vi "UHR-Fleezers Control (host) - 12.6.1.vi"() -> ()   [LabVIEW 2012] (continued)
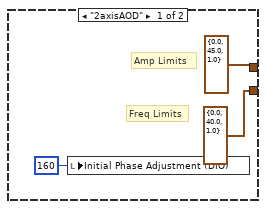
[diagram p2: hidden frame]
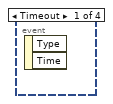
[diagram p3: hidden frame]
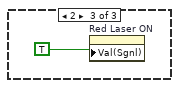
[diagram p6: hidden frame]
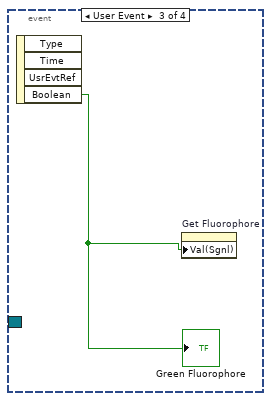
[diagram p7: hidden frame]
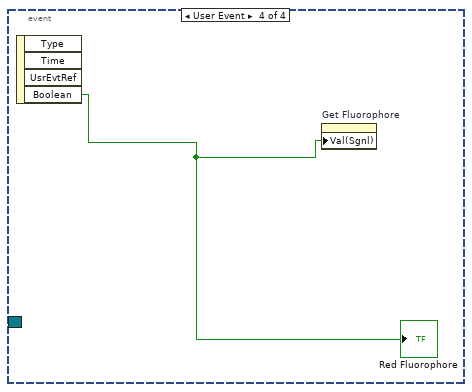
[diagram p8: hidden frame]
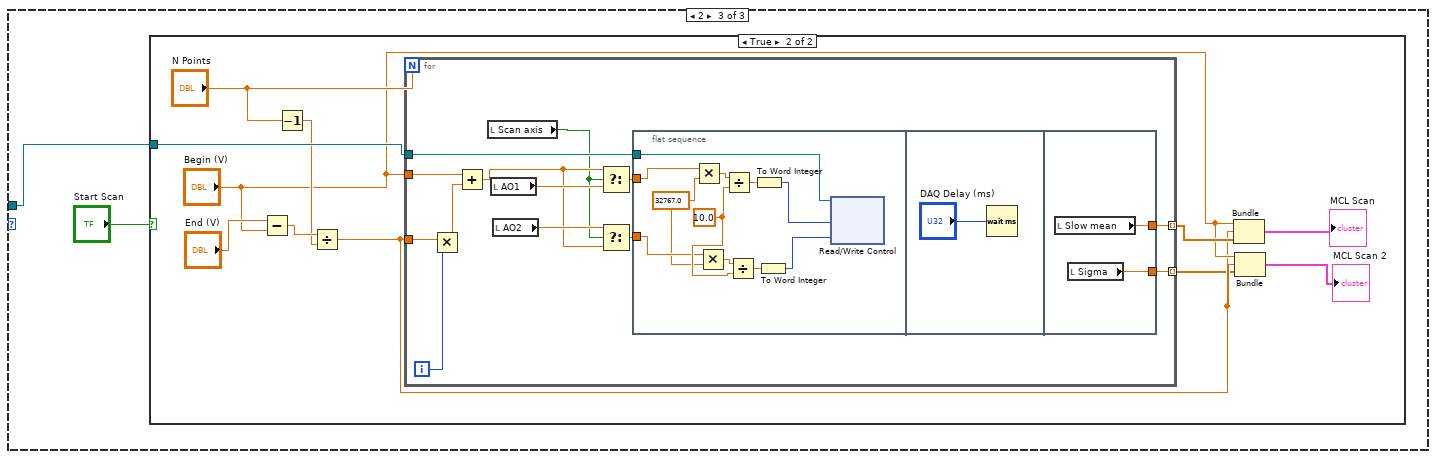
[diagram p10: hidden frame]
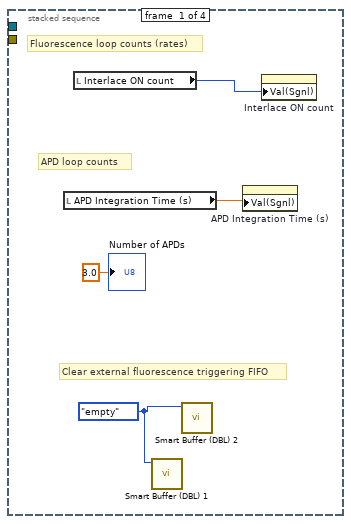
[diagram p12: hidden frame]
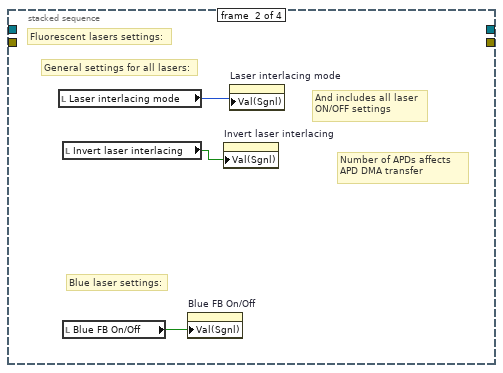
[diagram p13: hidden frame]
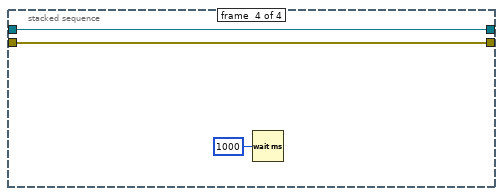
[diagram p14: hidden frame]
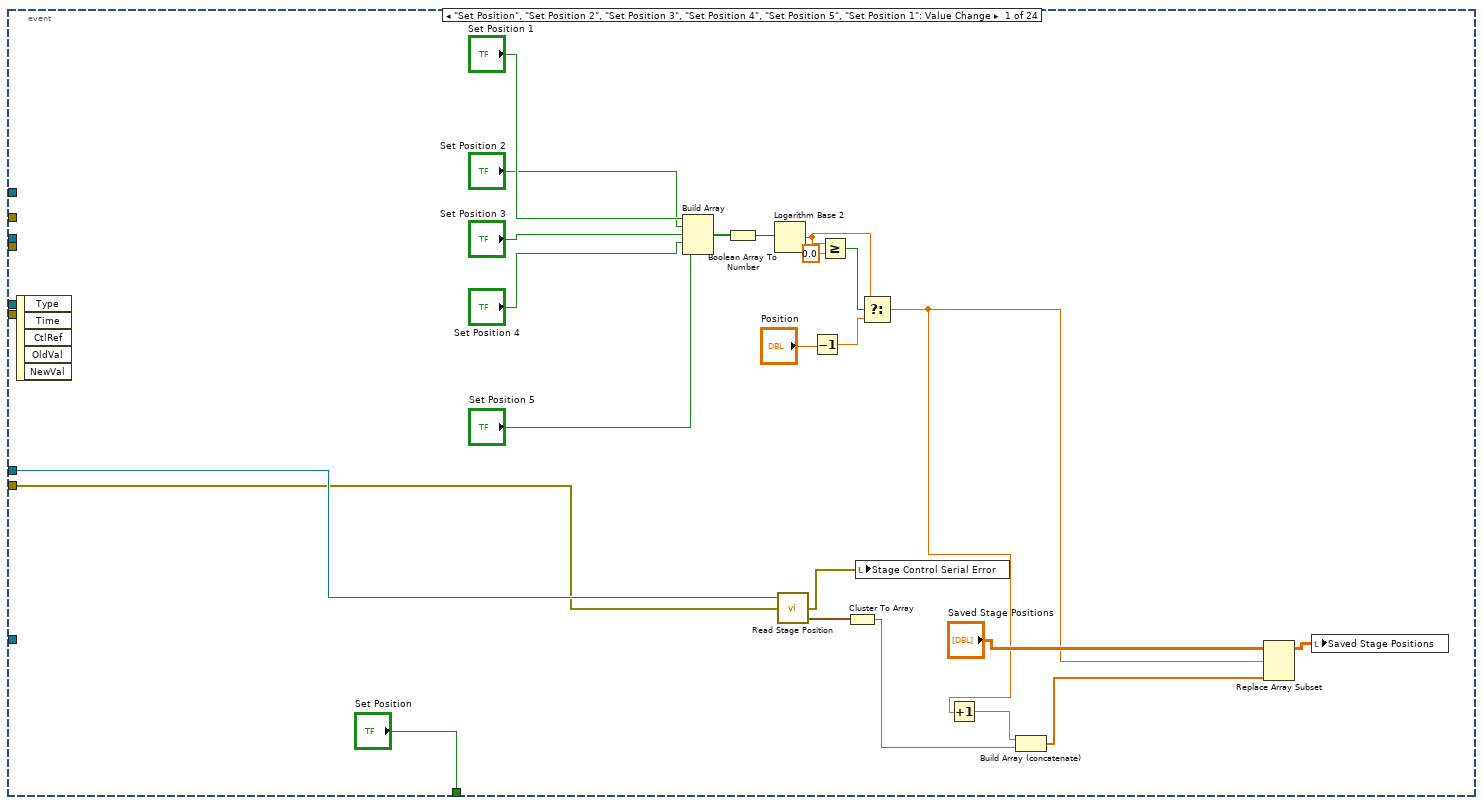
[diagram p16: hidden frame]
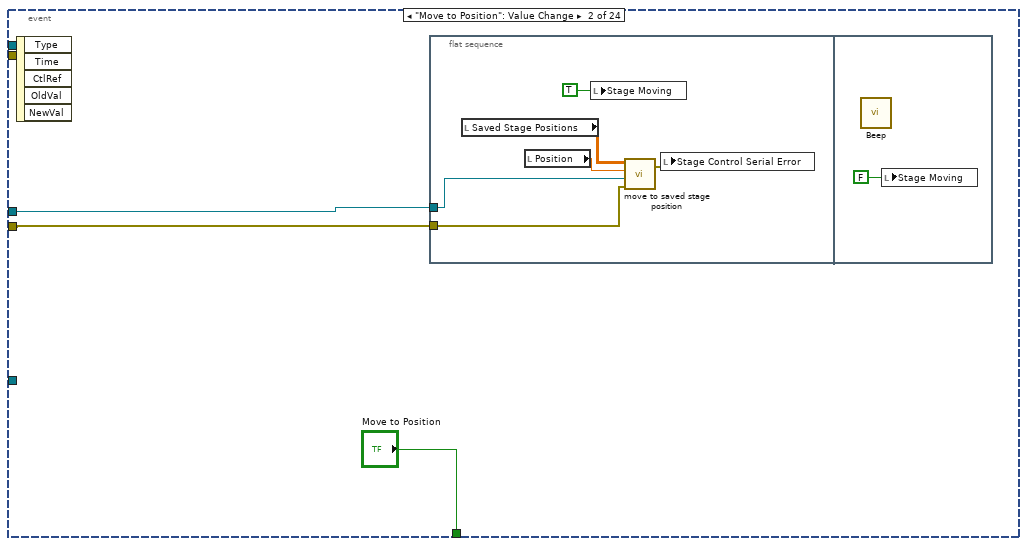
[diagram p17: hidden frame]
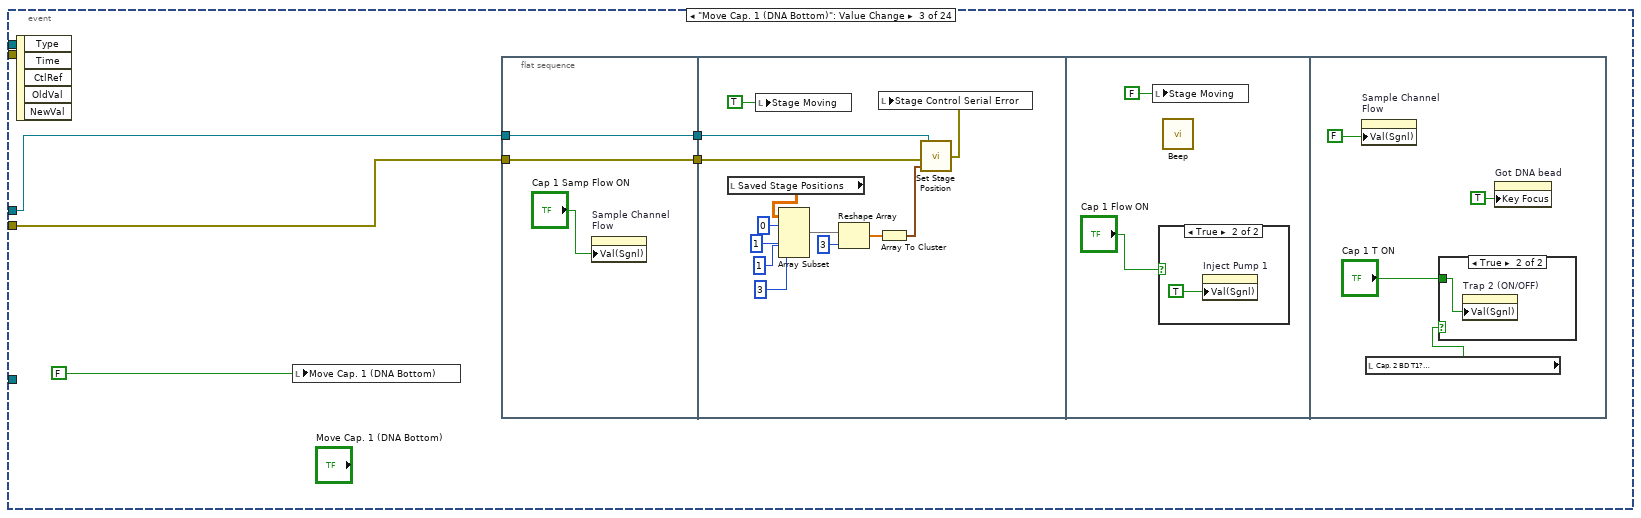
[diagram p18: hidden frame]
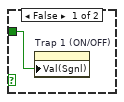
[diagram p20: hidden frame]
            n2987 = Build Array (concatenate)(w4589, w4590, w4587) -> (w4562:dbl[])
            n2988 = case "If fluorescence data to be saved" shown="True" w4579 {
              tunnel: w4563 -> [_ w4657]
              tunnel: [refnum<k0> refnum w4637] -> w4580
              frame False {
              }
              frame True {
                w4636 = 0.0
                n2989 = local read "APD Integration Time (s)"() -> (w4642:dbl)
                n2990 = local read "N APD Samp/step"() -> (w4635:dbl)
                n2991 = local read "Number of APDs"() -> (w4634:u8)
                n2992 = Path To String(path=w4657) -> (string=w4656:string)
                n2993 = String Length(string=w4656) -> (length=w4655:i32)
                n2994 = Subtract(x=w4655, y=4) -> (x-y=w4653:i32)
                n2995 = String Subset(string=w4656, length (rest)=w4653) -> (substring=w4652:string)  [unwired: 1 out]
                n2996 = Build Array(w4642, w4635, w4634, w4636, w4636, w4636, w4636, w4636) -> (w4639:dbl[])
                n2997 = Concatenate Strings(w4652, "_fl.dat" ("string")) -> (w4650:string)
                n2998 = Array Size(array=w4639) -> (size(s)=w4641:i32)
                n2999 = String To Path(string=w4650) -> (path=w4646:path)
                n3000 = Open/Create/Replace File(file path (use dialog)=w4646, operation (0:open)=T29."create", access (0:read/write)=enum16{"read/write", "read-only", "write-only"}."write-only") -> (refnum out=w4647:refnum<file>)  [unwired: 1 in, 4 out]
                n3001 = Deny Access(7:w4647) -> (3:w4643:refnum<file>)  [unwired: 1 in, 2 out]
                n3002 = To Double Precision Float(number=w4641) -> (double precision float=w4640:dbl)
                n3003 = Build Array (concatenate)(w4640, w4639) -> (w4638:dbl[])
                n3004 = Write to Binary File(file (use dialog)=w4643, data=w4638, 5:FALSE ("prepend array or string size? (T)"), 9:T28."big-endian, network order" ("byte order (0:big-endian, network order)")) -> (refnum out=w4637:refnum<file>)  [unwired: 1 in, 3 out]
              }
            }
            n3005 = case shown="True" w4567 {
              tunnel: w4563 -> [_ w4618]
              tunnel: [refnum<k0> refnum w4617] -> w4568
              frame False {
              }
              frame True {
                w4613 = 0.0 ("element")
                n3006 = Path To String(path=w4618) -> (string=w4632:string)
                n3007 = Build Array(w4613, w4613, w4613, w4613, w4613, w4613, w4613, w4613) -> (w4614:dbl[])
                n3008 = String Length(string=w4632) -> (length=w4631:i32)
                n3009 = Subtract(x=w4631, y=4) -> (x-y=w4629:i32)
                n3010 = Array Size(array=w4614) -> (size(s)=w4616:i32)
                n3011 = String Subset(string=w4632, length (rest)=w4629) -> (substring=w4628:string)  [unwired: 1 out]
                n3012 = To Double Precision Float(number=w4616) -> (double precision float=w4615:dbl)
                n3013 = Concatenate Strings(w4628, "_pos.dat" ("string")) -> (w4626:string)
                n3014 = Build Array (concatenate)(w4615, w4614) -> (w4612:dbl[])
                n3015 = String To Path(string=w4626) -> (path=w4622:path)
                n3016 = Open/Create/Replace File(file path (use dialog)=w4622, operation (0:open)=T29."create", access (0:read/write)=enum16{"read/write", "read-only", "write-only"}."write-only") -> (refnum out=w4623:refnum<file>)  [unwired: 1 in, 4 out]
                n3017 = Deny Access(7:w4623) -> (3:w4619:refnum<file>)  [unwired: 1 in, 2 out]
                n3018 = Write to Binary File(file (use dialog)=w4619, data=w4612, 5:FALSE ("prepend array or string size? (T)"), 9:T28."big-endian, network order" ("byte order (0:big-endian, network order)")) -> (refnum out=w4617:refnum<file>)  [unwired: 1 in, 3 out]
              }
            }
            n3019 = Write to Binary File(file (use dialog)=w4603, data=w4562, 5:w4585, 9:w4584) -> (refnum out=w4586:refnum<file>)  [unwired: 1 in, 3 out]
            n3020 = Write to Binary File(file (use dialog)=w4586, data="Comment (data description)", 5:w4585, 9:w4584) -> (refnum out=w4583:refnum<file>)  [unwired: 1 in, 3 out]
            n3021 = local read "connection reference"() -> (w4565:T17)
            n3022 = Bundle("Comment (data description)"="Comment (data description)", "Channel 1 Buffer"="Channel 1 Buffer", "Channel 2 Buffer"="Channel 2 Buffer", "Channel 3 Buffer"="Channel 3 Buffer", "Title"="Title", "DNA Construct"="DNA Construct", "Bead diameter"="Bead diameter", "Name"="Name") -> (w4553:T47)  [unwired: 1 in]
            n3023 = call "MattFileCreator-v9.vi"("Comments"=w4553, "Input Array"=w4562, "File path"=w4563, "table"="labview", "connection reference"=w4565) -> ("connection reference out"=w4564:T17)  [unwired: 5 in, 1 out]
            n3024 = local write "connection reference"(w4564) -> ()
          }
        }
        n3025 = feedback-in #27(w4513) -> ()
        n3026 = feedback-in #28(w4540) -> ()
        n3027 = feedback-in #29(w4512) -> ()
        n3028 = feedback-in #30(w4523) -> ()
        n3029 = feedback-in #31(w4526) -> ()
        n3030 = feedback-in #32(w4539) -> ()
        n3031 = feedback-in #33(w4529) -> ()
      }
      frame #1 {
        n3032 = local read "Saving..."() -> (w4783:bool)
        n3033 = case shown="True" w4783 {
          tunnel: w4787 -> [_ w4798]
          tunnel: w4786 -> [_ w4812]
          tunnel: w4785 -> [_ w4808]
          tunnel: w4784 -> [_ w4807]
          tunnel: w4782 -> [_ w4806]
          tunnel: w4781 -> [_ w4801]
          tunnel: w4780 -> [_ w4800]
          tunnel: w4779 -> [_ w4799]
          tunnel: w4778 -> [_ w4797]
          tunnel: w4777 -> [_ w4795]
          tunnel: w4776 -> [_ w4794]
          tunnel: w4775 -> [_ w4793]
          tunnel: w4774 -> [_ w4792]
          tunnel: w4773 -> [_ w4791]
          tunnel: w4772 -> [_ w4790]
          tunnel: w4771 -> [_ w4789]
          tunnel: w4770 -> [_ w4788]
          frame False {
          }
          frame True {
            n3034 = Multiply(x=w4798, y=w4797) -> (x*y=→"Time (s)":dbl)
            n3035 = Less Or Equal?(x=w4798, y=w4806) -> (x <= y?=w4810:bool)
            n3036 = Or(x="Stop Saving", y="Abort save 2") -> (x .or. y?=w4802:bool)
            n3037 = Not(x=w4802) -> (.not. x?=w4811:bool)
            n3038 = And(x=w4810, y=w4811) -> (x .and. y?=w4809:bool)
            n3039 = case shown="True" w4809 {
              tunnel: w4812 -> [w4819 w4910]
              tunnel: [0.0 w4913] -> w4805
              tunnel: w4798 -> [_ w4911]
              tunnel: w4806 -> [_ w4912]
              tunnel: w4808 -> [_ w4907]
              tunnel: w4807 -> [_ _]
              tunnel: w4801 -> [w4817 w4900]
              tunnel: w4800 -> [w4816 w4901]
              tunnel: w4799 -> [_ w4899]
              tunnel: w4795 -> [_ w4898]
              tunnel: w4794 -> [_ w4822]
              tunnel: w4793 -> [_ w4891]
              tunnel: w4792 -> [_ w4838]
              tunnel: w4791 -> [w4813 w4855]
              tunnel: w4790 -> [w4814 w4854]
              tunnel: w4789 -> [_ w4851]
              tunnel: w4788 -> [_ w4849]
              frame False {
                w4815 = FALSE
                n3040 = Close File(refnum=w4819) -> ()  [unwired: 1 in, 2 out]
                n3041 = case shown="True" w4816 {
                  tunnel: w4817 -> [_ w4821]
                  frame False {
                  }
                  frame True {
                    n3042 = Close File(refnum=w4821) -> ()  [unwired: 1 in, 2 out]
                  }
                }
                n3043 = case shown="True" w4813 {
                  tunnel: w4814 -> [_ w4820]
                  frame False {
                  }
                  frame True {
                    n3044 = Close File(refnum=w4820) -> ()  [unwired: 1 in, 2 out]
                  }
                }
                n3045 = local write "Raster Scanning..."(w4815) -> ()
                n3046 = local write "Calibrating Trap..."(w4815) -> ()
                n3047 = call <vilib>:"Beep.vi"() -> ()  [unwired: 3 in, 9 out]
                n3048 = local write "Stop Saving"(w4815) -> ()
                "Saving..." <- w4815
              }
              frame True {
                n3049 = local read "Calibrating Trap..."() -> (w4902:bool)
                n3050 = case "Write fl. data" shown="True" w4901 {
                  tunnel: w4900 -> [_ w4936]
                  tunnel: w4899 -> [_ w4935]
                  frame False {
                  }
                  frame True {
                    n3051 = Write to Binary File(file (use dialog)=w4936, data=w4935, 5:FALSE ("prepend array or string size? (T)"), 9:T28."big-endian, network order" ("byte order (0:big-endian, network order)")) -> ()  [unwired: 1 in, 4 out]
                  }
                }
                n3052 = Greater?(x="Save ave N", y=1.0) -> (0:w4905:bool)
                n3053 = Not(x=w4902) -> (.not. x?=w4904:bool)
                n3054 = And(x=w4904, y=w4905) -> (x .and. y?=w4852:bool)
                n3055 = case shown="True" w4852 {
                  tunnel: w4851 -> [w4916 w4927]
                  tunnel: [w4916 w4919] -> w4850
                  tunnel: "Save ave N" -> [_ w4920]
                  frame False {
                  }
                  frame True {
                    w4917 = 2 ("dimension size")
                    n3056 = Array Size(array=w4927) -> (size(s)=w4921:i32)
                    n3057 = Divide(x=w4921, y=w4917) -> (x/y=w4925:dbl)
                    n3058 = Reshape Array(w4927, w4925, w4917) -> (w4926:u64[][])
                    n3059 = Transpose 2D Array(2D array=w4926) -> (transposed array=w4924:u64[][])
                    n3060 = for {
                      tunnel: w4924 -> [w4929] mode=indexing
                      tunnel: [w4928] -> w4918 mode=indexing
                      tunnel: w4920 -> [w4930]
                      workers-P: _ -> [_]
                      n3061 = call "downsample 1D array - U64.vi"("Ave N"=w4930, "Array In"=w4929) -> ("Array Out"=w4928:u64[])  [unwired: 1 in]
                    }
                    n3062 = Transpose 2D Array(2D array=w4918) -> (transposed array=w4923:u64[][])
                    n3063 = Divide(x=w4921, y=w4920) -> (x/y=w4922:dbl)
                    n3064 = Reshape Array(w4923, w4922) -> (w4919:u64[])
                  }
                }
                n3065 = case shown="True" w4852 {
                  tunnel: w4907 -> [w4939 w4951]
                  tunnel: [w4939 w4943] -> w4903
                  tunnel: "Save ave N" -> [_ w4944]
                  tunnel: w4898 -> [_ w4942]
                  frame False {
                  }
                  frame True {
                    n3066 = Array Size(array=w4951) -> (size(s)=w4945:i32)
                    n3067 = Array Size(array=w4942) -> (size(s)=w4941:i32)
                    n3068 = Divide(x=w4945, y=w4941) -> (x/y=w4949:dbl)
                    n3069 = Reshape Array(w4951, w4949, w4941) -> (w4950:i16[][])
                    n3070 = Transpose 2D Array(2D array=w4950) -> (transposed array=w4948:i16[][])
                    n3071 = for {
                      tunnel: w4948 -> [w4954] mode=indexing
                      tunnel: [w4953] -> w4940 mode=indexing
                      tunnel: w4944 -> [w4952]
                      workers-P: _ -> [_]
                      n3072 = call "downsample 1D array - I16.vi"("Ave N"=w4952, "Array In"=w4954) -> ("Array Out"=w4953:i16[])  [unwired: 1 out]
                    }
                    n3073 = Transpose 2D Array(2D array=w4940) -> (transposed array=w4947:i16[][])
                    n3074 = Divide(x=w4945, y=w4944) -> (x/y=w4946:dbl)
                    n3075 = Reshape Array(w4947, w4946) -> (w4943:i16[])
                  }
                }
                n3076 = Index Array(array=w4838, index=2) -> (element=w4839:waveform(dbl))
                n3077 = Index Array(array=w4838, index=1) -> (element=w4872:waveform(dbl))
                n3078 = Index Array(array=w4838, index=0) -> (element=w4874:waveform(dbl))
                n3079 = Unbundle By Name(w4839) -> ("Y"=w4841:dbl[])
                n3080 = Unbundle By Name(w4872) -> ("Y"=w4876:dbl[])
                n3081 = Unbundle By Name(w4874) -> ("Y"=w4884:dbl[])
                n3082 = case "Write trap pos. data" shown="True" w4855 {
                  tunnel: w4854 -> [_ w4932]
                  tunnel: w4850 -> [_ w4931]
                  frame False {
                  }
                  frame True {
                    n3083 = Write to Binary File(file (use dialog)=w4932, data=w4931, 5:FALSE ("prepend array or string size? (T)"), 9:T28."big-endian, network order" ("byte order (0:big-endian, network order)")) -> ()  [unwired: 1 in, 4 out]
                  }
                }
                n3084 = Write to Binary File(file (use dialog)=w4910, data=w4903, 5:FALSE ("prepend array or string size? (T)"), 9:T28."big-endian, network order" ("byte order (0:big-endian, network order)")) -> ()  [unwired: 1 in, 4 out]
                n3085 = feedback #34(w4841) -> (w4842:dbl[])
                n3086 = Build Array (concatenate)(w4842, w4841) -> (w4837:dbl[])
                n3087 = Select(t=w4841, s=w4822, f=w4837) -> (s? t:f=w4827:dbl[])
                n3088 = feedback-in #34(w4827) -> ()
                n3089 = feedback #35(w4876) -> (w4878:dbl[])
                n3090 = Build Array (concatenate)(w4878, w4876) -> (w4877:dbl[])
                n3091 = Select(t=w4876, s=w4822, f=w4877) -> (s? t:f=w4866:dbl[])
                n3092 = feedback-in #35(w4866) -> ()
                n3093 = feedback #36(w4884) -> (w4897:dbl[])
                n3094 = Build Array (concatenate)(w4897, w4884) -> (w4896:dbl[])
                n3095 = Select(t=w4884, s=w4822, f=w4896) -> (s? t:f=w4871:dbl[])
                n3096 = feedback-in #36(w4871) -> ()
                n3097 = Divide(x=w4911, y=w4912) -> (x/y=w4914:dbl)
                n3098 = Multiply(x=w4914, y=100.0) -> (x*y=w4913:dbl)
                n3099 = Build Array(w4871, w4866, w4827) -> (→"Saved APD":dbl[][])
                n3100 = Array Size(array=w4871) -> (size(s)=w4889:i32)
                n3101 = Unbundle By Name(w4891) -> ("Y"=w4895:dbl[])
                n3102 = Subtract(x=w4889, y="N pts to average") -> (x-y=w4824:i32)
                n3103 = Multiply(x="N pts to average", y=u16 2) -> (x*y=w4867:u16)
                n3104 = Subtract(x=w4889, y=w4867) -> (x-y=w4825:i32)
                n3105 = feedback #37(w4895) -> (w4894:dbl[])
                n3106 = Build Array (concatenate)(w4894, w4895) -> (w4893:dbl[])
                n3107 = Select(t=w4895, s=w4822, f=w4893) -> (s? t:f=w4892:dbl[])
                "Trap Delta Graph" <- w4892
                n3108 = feedback-in #37(w4892) -> ()
                n3109 = Array Subset(array=w4871, index=w4824, length="N pts to average") -> (w4888:dbl[])
                n3110 = Array Subset(array=w4871, index=w4825, length="N pts to average") -> (w4887:dbl[])
                n3111 = Array Subset(array=w4866, index=w4824, length="N pts to average") -> (w4869:dbl[])
                n3112 = Array Subset(array=w4866, index=w4825, length="N pts to average") -> (w4868:dbl[])
                n3113 = Array Subset(array=w4827, index=w4824, length="N pts to average") -> (w4836:dbl[])
                n3114 = Array Subset(array=w4827, index=w4825, length="N pts to average") -> (w4835:dbl[])
                n3115 = Index Array(array=w4849, index=0) -> (element=w4847:waveform(dbl))
                n3116 = call-poly <vilib>:"Mean.vi"("X"=w4888) -> ("mean"=w4886:dbl)  [unwired: 1 out]
                n3117 = call-poly <vilib>:"Mean.vi"("X"=w4869) -> ("mean"=w4865:dbl)  [unwired: 1 out]
                n3118 = call-poly <vilib>:"Mean.vi"("X"=w4887) -> ("mean"=w4885:dbl)  [unwired: 1 out]
                n3119 = call-poly <vilib>:"Mean.vi"("X"=w4868) -> ("mean"=w4864:dbl)  [unwired: 1 out]
                n3120 = call-poly <vilib>:"Mean.vi"("X"=w4836) -> ("mean"=w4834:dbl)  [unwired: 1 out]
                n3121 = call-poly <vilib>:"Mean.vi"("X"=w4835) -> ("mean"=w4833:dbl)  [unwired: 1 out]
                n3122 = Unbundle By Name(w4847) -> ("Y"=w4845:dbl[])
                n3123 = Subtract(x=w4865, y=w4864) -> (x-y=w4856:dbl)
                "Delta Fl. 2" <- w4856
                n3124 = Subtract(x=w4834, y=w4833) -> (x-y=w4828:dbl)
                "Delta Fl. 3" <- w4828
                n3125 = Subtract(x=w4886, y=w4885) -> (x-y=w4883:dbl)
                "Delta Fl. 1" <- w4883
                n3126 = feedback #38(w4845) -> (w4844:dbl[])
                n3127 = Build Array (concatenate)(w4844, w4845) -> (w4846:dbl[])
                n3128 = Initialize Array(w4883, 1 ("dimension size")) -> (w4880:dbl[])
                n3129 = Initialize Array(w4856, 1 ("dimension size")) -> (w4861:dbl[])
                n3130 = Initialize Array(w4828, 1 ("dimension size")) -> (w4830:dbl[])
                n3131 = Select(t=w4845, s=w4822, f=w4846) -> (s? t:f=w4843:dbl[])
                "Saved trap pos" <- w4843
                n3132 = feedback-in #38(w4843) -> ()
                n3133 = feedback #39(w4880) -> (w4881:dbl[])
                n3134 = Build Array (concatenate)(w4881, w4880) -> (w4879:dbl[])
                n3135 = feedback #40(w4861) -> (w4862:dbl[])
                n3136 = feedback #41(w4830) -> (w4831:dbl[])
                n3137 = Build Array (concatenate)(w4862, w4861) -> (w4860:dbl[])
                n3138 = Build Array (concatenate)(w4831, w4830) -> (w4829:dbl[])
                n3139 = Select(t=w4880, s=w4822, f=w4879) -> (s? t:f=w4859:dbl[])
                n3140 = feedback-in #39(w4859) -> ()
                n3141 = Select(t=w4861, s=w4822, f=w4860) -> (s? t:f=w4858:dbl[])
                n3142 = feedback-in #40(w4858) -> ()
                n3143 = Select(t=w4830, s=w4822, f=w4829) -> (s? t:f=w4823:dbl[])
                n3144 = feedback-in #41(w4823) -> ()
                n3145 = Build Array(w4859, w4858, w4823) -> (→"Save APD Deriv":dbl[][])
              }
            }
            "Progress" <- w4805
            "Progress 2" <- w4805
          }
        }
      }
    }
    n3146 = local read "wait to reset values"() -> (w3456:bool)
    n3147 = Not(x=w3454) -> (.not. x?=w3457:bool)
    n3148 = And(x=w3457, y=w3456) -> (x .and. y?=w3458:bool)
    n3149 = case "Part of MCL raster scanning: returns to initial positions after scan done" shown="True" w3458 {
      tunnel: w3189 -> [w4333 w4340]
      tunnel: [w4333 w4339] -> w3460
      tunnel: w3188 -> [w4332 w4338]
      tunnel: [w4332 w4337] -> w3455
      frame False {
      }
      frame True {
        w4348 = 10.0 ("y")
        w4347 = 32767.0 ("y")
        # "to return scan values\nafter a synchronous \nAOM scan"
        n3150 = local read "AO2"() -> (w4341:dbl)
        n3151 = local read "AO1"() -> (w4342:dbl)
        n3152 = local write "wait to reset values"(FALSE ("wait to reset values")) -> ()
        n3153 = Multiply(x=w4342, y=w4347) -> (x*y=w4344:dbl)
        n3154 = Multiply(x=w4341, y=w4347) -> (x*y=w4346:dbl)
        n3155 = Divide(x=w4344, y=w4348) -> (x/y=w4343:dbl)
        n3156 = Divide(x=w4346, y=w4348) -> (x/y=w4345:dbl)
        n3157 = To Word Integer(number=w4343) -> (16bit integer=w4349:i16)
        n3158 = To Word Integer(number=w4345) -> (16bit integer=w4350:i16)
        n3159 = local read "Total Counts (ticks)"() -> (w4334:u16)
        n3160 = xnode "Read/Write Control"("FPGA VI Reference In"=w4340, "error in"=w4338, "AO1"=w4349, "AO2"=w4350, "MCL count"=w4334) -> ("FPGA VI Reference Out"=w4339:T20, "error out"=w4337:errorcluster)
        n3161 = local read "Scan Range (V)\n(of steps)"() -> (w4335:dbl)
        n3162 = property on="Scan Range (V)\n(of steps)" class="DigNum (strict)"("Val(Sgnl)"=w4335) -> ()  [unwired: 2 in, 2 out]
      }
    }
    n3163 = node-c288() -> ()  [unwired: 2 out]
  }
  n3164 = flat-sequence "Video" {
    tunnel: [w4964] -> w115
    tunnel: w115 -> [w5004]
    frame #0 {
      n3165 = while {
        stop <- w4956 continue-if-true
        n3166 = call "Close Video Capture.vi"() -> ("error code OUT"=w4958:i32)
        n3167 = Equal?(x=w4958, y=0) -> (x = y?=w4956:bool)
      }
      n3168 = local write "Stop All"(FALSE ("Stop All")) -> ()
    }
    frame #1 {
      n3169 = call "DMR_Init.vi"() -> ()  [unwired: 3 out]
    }
    frame #2 {
      w4959 = "DE245428202"  # MSU fleezers card #
      (unwired) "DE019116701"  # Illinois fleezers card #
      # "Setting the destination format to Mono8 makes sure that the image can be displayed in the intensity plot."
      n3170 = call "DMR_GetDevice.vi"("search string IN"=w4959) -> ("device handle OUT"=w4982:i32)  [unwired: 4 in, 2 out]
      n3171 = call "DMR_OpenDevice.vi"("device handle IN"=w4982) -> ("driver handle OUT"=w4965:i32)  [unwired: 4 out]
      n3172 = call "DMR_FindList.vi"("flags IN"=u32 0 ("flags"), "list name IN"="" ("String"), "list type IN"=T48."camera descriptions", "driver handle IN"=w4965) -> ("list handle OUT"=w4968:i32)  [unwired: 2 out]
      n3173 = call "DMR_FindList.vi"("flags IN"=u32 0 ("flags"), "list name IN"="Base", "list type IN"=T48."setting", "driver handle IN"=w4965) -> ("list handle OUT"=w4966:i32)  [unwired: 2 out]
      n3174 = call "OBJ_GetHandle.vi"("object name IN"="VideoStandard", "list handle IN"=w4968) -> ("object handle OUT"=w4962:i32)  [unwired: 3 out]
      n3175 = call "OBJ_GetHandle.vi"("object name IN"="PixelFormat", "list handle IN"=w4966) -> ("object handle OUT"=w4976:i32)  [unwired: 3 out]
      n3176 = call "OBJ_SetS.vi"("value index IN"=0, "value IN"="NTSC M", "object handle IN"=w4962) -> ()  [unwired: 2 out]
      n3177 = call "OBJ_SetS.vi"("value index IN"=0, "value IN"="Mono8" ("value"), "object handle IN"=w4976) -> ()  [unwired: 2 out]
      n3178 = call "OBJ_GetHandle.vi"("object name IN"="VideoChannel", "list handle IN"=w4966) -> ("object handle OUT"=w4972:i32)  [unwired: 3 out]
      n3179 = while {
        tunnel: [w4986] -> w4964
        tunnel: w4965 -> [w4983]
        stop <- w4984 continue-if-true
        n3180 = call "DMR_ImageRequestSingle.vi"("request control IN"=0, "driver handle IN"=w4983) -> ("error code OUT"=w4985:i32, "driver handle OUT"=w4986:i32)  [unwired: 2 out]
        n3181 = Equal To 0?(x=w4985) -> (x = 0?=w4984:bool)
      }
      n3182 = call "OBJ_SetI.vi"("value index IN"=0, "value IN"=3 ("Video channel"), "object handle IN"=w4972) -> ()  [unwired: 2 out]
    }
    frame #3 {
      w4992 = T18 0 items=["Grayscale (U8)", "Grayscale (I16)", "Grayscale (SGL)", "Complex (CSG)", "RGB (U32)", "HSL (U32)", "RGB (U64)"] ("Image Type")
      w5000 = T18 0 items=["Grayscale (U8)", "Grayscale (I16)", "Grayscale (SGL)", "Complex (CSG)", "RGB (U32)", "HSL (U32)", "RGB (U64)"] ("Image Type")
      n3183 = for "Create Greyscale map" {
        N: 256 -> [_]
        tunnel: [w5006] -> w4989 mode=indexing
        workers-P: _ -> [_]
        i -> [w5009]
        n3184 = To Unsigned Byte Integer(number=w5009) -> (unsigned 8bit integer=w5005:u8)
        n3185 = Join Numbers(hi=w5005, lo=w5005) -> ((hi.lo)=w5008:u16)
        n3186 = Join Numbers(hi=w5005, lo=w5005) -> ((hi.lo)=w5007:u16)
        n3187 = Join Numbers(hi=w5008, lo=w5007) -> ((hi.lo)=w5006:u32)
      }
      n3188 = call "IMAQ Create"("Image Name"="Scaled video", "Image Type"=w4992) -> ("New Image"=w4991:T2)  [unwired: 2 in, 2 out]
      n3189 = call "IMAQ Create"("Image Name"="Main video", "Image Type"=w5000) -> ("New Image"=w5001:T2)  [unwired: 2 in, 2 out]
      n3190 = node-c288(0 ("Processor")) -> (w4999:T23)  [unwired: 3 out]
      n3191 = Initialize Array(u32 0 ("Window Number (0...15)"), 480 ("dimension size"), 640 ("dimension size")) -> (w4994:u32[][])
      n3192 = timed-loop {
        tunnel: w5004 -> [w5026]
        tunnel: [w5025] -> w5003
        tunnel: w5001 -> [w5024]
        timing: w4999 -> [_]
        timing-out: [_] -> w4998
        tunnel: w4994 -> [w5013]
        tunnel: w4991 -> [w5011]
        tunnel: w4989 -> [w5010]
        stop <- w5012 stop-if-true
        # "This block performs the \nactual image capture."
        n3193 = node-c288() -> ()  [unwired: 2 out]
        n3194 = local read "Stop All"() -> (w5012:bool)
        n3195 = Reciprocal(x="Video Capture Rate (Hz)") -> (1/x=w5016:dbl)
        n3196 = Multiply(x=w5016, y=1000.0) -> (x*y=w5014:dbl)
        n3197 = call "DMR_ImageRequestWaitFor.vi"("queue number IN"=0, "timeout(ms) IN"=500, "driver handle IN"=w5026) -> ("error code OUT"=w5030:i32, "request number OUT"=w5027:i32, "driver handle OUT"=w5028:i32)
        n3198 = feedback #42(T49 refnum ("Avi Refnum")) -> (w5018:T49)
        n3199 = case shown="True" "New Video File" {
          tunnel: [T49 refnum ("Avi Refnum") w5047] -> w5020
          tunnel: [FALSE TRUE] -> w5021
          tunnel: w5018 -> [_ w5043]
          frame False {
          }
          frame True {
            n3200 = call "Create new save file.vi"("Ext"=".avi" ("string"), "Index In"="Video Index") -> ("Path Out"=w5039:path, "Index Out"=w5040:dbl)  [unwired: 1 in]
            "Path Out" <- w5039
            n3201 = Not Equal?(x=w5043, y=T49 refnum ("Avi Refnum")) -> (x != y?=w5044:bool)
            n3202 = Increment(x=w5040) -> (x+1=w5049:dbl)
            n3203 = case shown="True" w5044 {
              tunnel: w5043 -> [_ w5050]
              frame False {
              }
              frame True {
                n3204 = call "IMAQ AVI Close"("Avi Refnum"=w5050) -> ()  [unwired: 1 in, 10 out]
              }
            }
            n3205 = local write "Video Index"(w5049) -> ()
            n3206 = call "IMAQ AVI Create"("Frames Per Second"=u32 30, "AVI Path"=w5039) -> ("Avi Refnum"=w5047:T49)  [unwired: 5 in, 4 out]
          }
        }
        n3207 = Equal To 0?(x=w5030) -> (x = 0?=w5029:bool)
        n3208 = Select(t=w5020, s=w5021, f=w5018) -> (s? t:f=w5019:T49)
        n3209 = feedback-in #42(w5019) -> ()
        n3210 = case shown="True" w5029 {
          tunnel: w5028 -> [w5051 w5085]
          tunnel: w5027 -> [_ w5084]
          tunnel: [w5051 w5081] -> w5025
          tunnel: w5024 -> [_ w5066]
          tunnel: w5013 -> [_ w5070]
          tunnel: w5019 -> [_ w5068]
          tunnel: w5011 -> [_ w5063]
          tunnel: w5010 -> [_ w5062]
          frame False {
          }
          frame True {
            w5075 = u32 0 ("X-offset IN")
            n3211 = call "DMR_GetImageRequestBufferData.vi"("driver handle IN"=w5085, "request number IN"=w5084) -> ("width OUT"=w5074:i32, "height OUT"=w5073:i32, "driver handle OUT"=w5080:i32, "request number OUT"=w5079:i32, "bytes per pixel OUT"=w5076:i32)  [unwired: 13 out]
            n3212 = call "DMR_GetImageRequestBufferImageData.vi"("driver handle IN"=w5080, "request number IN"=w5079, "bytes per pixel IN"=w5076, "X-offset IN"=w5075, "Y-offset IN"=w5075, "height IN"=w5073, "width IN"=w5074) -> ("driver handle OUT"=w5078:u32, "request number OUT"=w5077:u32, "image OUT"=w5055:u32[][])  [unwired: 10 out]
            n3213 = Transpose 2D Array(2D array=w5055) -> (transposed array=w5061:u32[][])
            n3214 = Select(t=w5061, s="Flip Y (or X)", f=w5055) -> (s? t:f=w5060:u32[][])
            n3215 = call "DMR_ImageRequestUnlock.vi"("request number IN"=w5077, "driver handle IN"=w5078) -> ("driver handle OUT"=w5083:i32)  [unwired: 1 in, 2 out]
            n3216 = for {
              tunnel: w5060 -> [w5120] mode=indexing
              tunnel: [w5119] -> w5058 mode=indexing
              n3217 = Reverse 1D Array(array=w5120) -> (reversed array=w5119:u32[])
            }
            n3218 = call "DMR_ImageRequestSingle.vi"("request control IN"=0, "driver handle IN"=w5083) -> ("driver handle OUT"=w5081:i32)  [unwired: 3 out]
            n3219 = Transpose 2D Array(2D array=w5058) -> (transposed array=w5059:u32[][])
            n3220 = Select(t=w5059, s="Flip Y (or X)", f=w5058) -> (s? t:f=w5056:u32[][])
            n3221 = Select(t=w5056, s="Flip Image", f=w5055) -> (s? t:f=w5053:u32[][])
            n3222 = case shown="True" "Averaging" {
              tunnel: w5053 -> [w5123 w5128]
              tunnel: [w5123 w5127] -> w5067
              tunnel: w5070 -> [_ w5125]
              frame False {
              }
              frame True {
                (unwired) 1
                w5133 = 1
                n3223 = feedback #43(w5125) -> (w5124:u32[][])
                n3224 = Add(x=w5128, y=w5124) -> (x+y=w5129:u32[][])
                n3225 = Select(t=w5125, s="Reset Averaging", f=w5129) -> (s? t:f=w5131:u32[][])
                n3226 = feedback-in #43(w5131) -> ()
                n3227 = feedback #44(w5133) -> (w5126:i32)
                n3228 = Divide(x=w5129, y=w5126) -> (x/y=w5130:dbl[][])
                n3229 = Increment(x=w5126) -> (x+1=w5134:i32)
                n3230 = To Unsigned Long Integer(number=w5130) -> (unsigned 32bit integer=w5127:u32[][])
                n3231 = Select(t=w5133, s="Reset Averaging", f=w5134) -> (s? t:f=w5132:i32)
                n3232 = feedback-in #44(w5132) -> ()
              }
            }
            n3233 = case shown="True" "Zoom video window" {
              tunnel: w5067 -> [_ w5099]
              tunnel: w5063 -> [_ w5098]
              frame False {
              }
              frame True {
                n3234 = To Double Precision Float(number=w5099) -> (double precision float=w5096:dbl[][])
                n3235 = In Range and Coerce(upper limit="Intensity Upper", x=w5096, lower limit="Intensity Lower") -> (coerced(x)=w5095:dbl[][])  [unwired: 1 out]
                n3236 = Subtract(x="Intensity Upper", y="Intensity Lower") -> (x-y=w5092:dbl)
                n3237 = Subtract(x=w5095, y="Intensity Lower") -> (x-y=w5093:dbl[][])
                n3238 = Divide(x=w5093, y=w5092) -> (x/y=w5094:dbl[][])
                n3239 = Multiply(x=255.0, y=w5094) -> (x*y=w5090:dbl[][])
                n3240 = To Unsigned Byte Integer(number=w5090) -> (unsigned 8bit integer=w5097:u8[][])
                n3241 = call "IMAQ ArrayToImage"("Image Pixels (U8)"=w5097, "Image"=w5098) -> ("Image Out"=w5086:T2)  [unwired: 4 in, 5 out]
                n3242 = First Call?() -> (First Call?: T/F=w5087:bool)
                n3243 = case shown="True" w5087 {
                  tunnel: w5086 -> [w5100 w5111]
                  frame False {
                    n3244 = flat-sequence {
                      tunnel: w5100 -> [w5106]
                      frame #0 {
                        w5103 = FALSE ("Get/Set Status? (Set)")
                        w5102 = 0 ("Window Number (0...15)")
                        n3245 = call "IMAQ WindSize"("Get/Set Status? (Set)"=w5103, "Window Number"=w5102) -> ("Width & Height out"=→"Window Size":cluster{"Width":i32, "Height":i32})  [unwired: 4 in, 2 out]
                        n3246 = call "IMAQ WindMove"("Window Number (0...15)"=w5102, "Get/Set Status? (Set)"=w5103) -> ("Coordinates (screen)"=→"Window Position":cluster{"X Position":i32, "Y Position":i32})  [unwired: 3 in, 1 out]
                        n3247 = call "IMAQ WindDraw"("Resize to Image Size? (Y)"=FALSE, "Window Number (0...15)"=w5102, "Image"=w5106) -> ()  [unwired: 7 in, 2 out]
                      }
                      frame #1 {
                        n3248 = call "IMAQ WindZoom 2"("Center Point"="Center Point", "Zoom to Fit? (False)"=FALSE, "Zoom Factor"="Zoom Factor") -> ()  [unwired: 5 in, 4 out]
                      }
                    }
                  }
                  frame True {
                    n3249 = flat-sequence {
                      tunnel: w5111 -> [w5114]
                      tunnel: [w5112] -> w5110
                      tunnel: w5110 -> [w5116]
                      frame #0 {
                        w5113 = TRUE ("Resize to Image Size? (Y)")
                        w5112 = 0 ("Window Number (0...15)")
                        n3250 = call "IMAQ WindNonTearing"("Window Number"=w5112, "NonTearing? (True)"=w5113) -> ()  [unwired: 8 in, 2 out]
                        n3251 = call "IMAQ WindDraw"("Resize to Image Size? (Y)"=w5113, "Window Number (0...15)"=w5112, "Image"=w5114) -> ()  [unwired: 7 in, 2 out]
                      }
                      frame #1 {
                        n3252 = call "IMAQ WindSize"("Scrollbars? (N)"=FALSE, "Width & Height"="Initial Window Size", "Window Number"=w5116) -> ()  [unwired: 3 in, 3 out]
                        n3253 = call "IMAQ WindMove"("Window Number (0...15)"=w5116, "Coordinates (screen)"="Initial Window Position") -> ()  [unwired: 3 in, 2 out]
                      }
                    }
                  }
                }
              }
            }
            n3254 = To Unsigned Byte Integer(number=w5067) -> (unsigned 8bit integer=w5065:u8[][])
            n3255 = call "IMAQ ArrayToImage"("Image Pixels (U8)"=w5065, "Image"=w5066) -> ("Image Out"=w5064:T2)  [unwired: 4 in, 5 out]
            "Primary Video Display" <- w5064
            n3256 = case shown="True" "Save Video" {
              tunnel: w5068 -> [_ w5122]
              tunnel: w5064 -> [_ w5121]
              frame False {
              }
              frame True {
                n3257 = call "IMAQ AVI Write Frame"("Image"=w5121, "Avi Refnum"=w5122) -> ()  [unwired: 2 in, 8 out]
              }
            }
            n3258 = case shown="True" "Save Image" {
              tunnel: w5065 -> [_ w5137]
              tunnel: w5062 -> [_ w5136]
              frame False {
              }
              frame True {
                n3259 = call <vilib>:"Flatten Pixmap.vi"("colors"=w5136, "8-bit pixmap"=w5137) -> ("image data"=w5143:T50)  [unwired: 4 in, 5 out]
                n3260 = call "Create new save file.vi"("Insert"="video_frame_" ("string"), "Ext"=".bmp" ("string"), "Index In"="Image Index") -> ("Path Out"=w5139:path, "Index Out"=w5144:dbl)
                n3261 = Increment(x=w5144) -> (x+1=w5138:dbl)
                n3262 = local write "Image Index"(w5138) -> ()
                n3263 = call <vilib>:"Write BMP File.vi"("image data"=w5143, "path to BMP file"=w5139) -> ()  [unwired: 1 in, 9 out]
              }
            }
          }
        }
        n3264 = node-c288(w5014) -> ()  [unwired: 1 out]
      }
      n3265 = node-c288(w4998) -> ()  [unwired: 1 out]
      n3266 = call "DMR_CloseDevice.vi"("driver handle IN"=w5003) -> ()  [unwired: 1 in, 4 out]
    }
    frame #4 {
      n3267 = call "DMR_Close.vi"() -> ()  [unwired: 1 out]
    }
  }
  n3268 = timed-loop "Rough control of MCL mirror stage (debugging)" {
    tunnel: w17 -> [w5151]
    tunnel: [w5150] -> w255
    timing: w11 -> [_]
    timing-out: [_] -> w10
    stop <- w5150 stop-if-true
    n3269 = node-c288() -> ()  [unwired: 2 out]
    n3270 = case shown="1" "MCL Mode" {
      tunnel: w5151 -> [_ w5154 w5201]
      frame 0, Default {
      }
      frame 1 {
        n3271 = node-c288() -> (w5156:T23)  [unwired: 4 out]
        n3272 = timed-loop "Oscillate MCL mirror" {
          timing: w5156 -> [_]
          timing-out: [_] -> w5155
          tunnel: w5154 -> [w5195]
          i -> [w5194]
          stop <- w5157 stop-if-true
          n3273 = node-c288() -> (w5193:i64)  [unwired: 1 out]
          n3274 = Multiply(x="AO1", y=32767.0) -> (x*y=w5189:dbl)
          n3275 = Multiply(x="AO2", y=32767.0) -> (x*y=w5184:dbl)
          n3276 = Divide(x=w5189, y=10.0) -> (x/y=w5190:dbl)
          n3277 = Divide(x=w5184, y=10.0) -> (x/y=w5185:dbl)
          n3278 = To Word Integer(number=w5190) -> (16bit integer=w5182:i16)
          n3279 = To Word Integer(number=w5185) -> (16bit integer=w5181:i16)
          n3280 = Divide(x=w5193, y=i64 1000) -> (x/y=w5164:dbl)
          n3281 = Multiply(x=w5164, y=w5194) -> (x*y=w5175:dbl)
          n3282 = Multiply(x="Osc. freq. (Hz) 2", y=6.283185307179586) -> (x*y=w5176:dbl)
          n3283 = Multiply(x=w5176, y=w5175) -> (x*y=w5174:dbl)
          n3284 = Sine(x=w5174) -> (sin(x)=w5173:dbl)
          n3285 = Multiply(x=w5173, y="Osc. amp. (V)") -> (x*y=w5171:dbl)
          n3286 = Add(x=w5171, y="Osc. center (V)") -> (x+y=w5169:dbl)
          n3287 = Divide(x=w5169, y=10.0) -> (x/y=w5167:dbl)
          n3288 = Multiply(x=w5167, y=32767.0) -> (x*y=w5162:dbl)
          n3289 = Select(t=w5162, s="Scan axis", f=w5182) -> (s? t:f=w5180:dbl)
          n3290 = Select(t=w5181, s="Scan axis", f=w5162) -> (s? t:f=w5179:dbl)
          n3291 = local read "MCL Mode"() -> (w5161:u16)
          n3292 = Not Equal?(x=w5161, y=u16 1) -> (x != y?=w5158:bool)
          n3293 = local read "Stop All"() -> (w5159:bool)
          n3294 = xnode "Read/Write Control"("FPGA VI Reference In"=w5195, "AO1"=w5180, "AO2"=w5179) -> ()  [unwired: 1 in, 2 out]
          n3295 = Compound Arithmetic op=OR(w5159, w5158) -> (w5157:bool)
          n3296 = node-c288() -> ()  [unwired: 2 out]
        }
        n3297 = node-c288(w5155) -> ()  [unwired: 1 out]
      }
      frame 2 {
        n3298 = case shown="True" "Start Scan" {
          tunnel: w5201 -> [_ w5213]
          frame False {
          }
          frame True {
            n3299 = Subtract(x="End (V)", y="Begin (V)") -> (x-y=w5209:dbl)
            n3300 = Decrement(x="N Points") -> (x-1=w5208:dbl)
            n3301 = Divide(x=w5209, y=w5208) -> (x/y=w5206:dbl)
            n3302 = for {
              N: "N Points" -> [_]
              tunnel: "Begin (V)" -> [w5226]
              tunnel: w5213 -> [w5218]
              tunnel: [w5217] -> w5212 mode=indexing
              tunnel: w5206 -> [w5216]
              tunnel: [w5214] -> w5205 mode=indexing
              i -> [w5225]
              n3303 = Multiply(x=w5216, y=w5225) -> (x*y=w5224:dbl)
              n3304 = Add(x=w5226, y=w5224) -> (x+y=w5221:dbl)
              n3305 = local read "Scan axis"() -> (w5215:bool)
              n3306 = local read "AO1"() -> (w5223:dbl)
              n3307 = local read "AO2"() -> (w5222:dbl)
              n3308 = Select(t=w5221, s=w5215, f=w5223) -> (s? t:f=w5220:dbl)
              n3309 = Select(t=w5222, s=w5215, f=w5221) -> (s? t:f=w5219:dbl)
              n3310 = flat-sequence {
                tunnel: w5220 -> [w5230]
                tunnel: w5219 -> [w5229]
                tunnel: w5218 -> [w5227]
                tunnel: [w5240] -> w5217
                tunnel: [w5239] -> w5214
                frame #0 {
                  w5233 = 10.0 ("y")
                  w5228 = 32767.0 ("y")
                  n3311 = Multiply(x=w5230, y=w5228) -> (x*y=w5236:dbl)
                  n3312 = Multiply(x=w5229, y=w5228) -> (x*y=w5234:dbl)
                  n3313 = Divide(x=w5236, y=w5233) -> (x/y=w5237:dbl)
                  n3314 = Divide(x=w5234, y=w5233) -> (x/y=w5235:dbl)
                  n3315 = To Word Integer(number=w5237) -> (16bit integer=w5231:i16)
                  n3316 = To Word Integer(number=w5235) -> (16bit integer=w5232:i16)
                  n3317 = xnode "Read/Write Control"("FPGA VI Reference In"=w5227, "AO1"=w5231, "AO2"=w5232) -> ()  [unwired: 1 in, 2 out]
                }
                frame #1 {
                  n3318 = Wait (ms)(milliseconds to wait="DAQ Delay (ms)") -> ()  [unwired: 1 out]
                }
                frame #2 {
                  n3319 = local read "Slow mean"() -> (w5240:dbl)
                  n3320 = local read "Sigma"() -> (w5239:dbl)
                }
              }
            }
            n3321 = Bundle("Begin (V)"="Begin (V)", w5206, w5212) -> (→"MCL Scan":cluster{"Begin (V)":dbl, dbl, dbl[]})  [unwired: 1 out]
            n3322 = Bundle("Begin (V)"="Begin (V)", w5206, w5205) -> (→"MCL Scan 2":cluster{"Begin (V)":dbl, dbl, dbl[]})  [unwired: 1 out]
          }
        }
      }
    }
    n3323 = local read "Stop All"() -> (w5150:bool)
    n3324 = node-c288() -> ()  [unwired: 2 out]
  }
  n3325 = node-c288(w10) -> ()  [unwired: 1 out]
  n3326 = node-c288(w126) -> ()  [unwired: 1 out]
  n3327 = node-c288(w128) -> ()  [unwired: 1 out]
  n3328 = property on="Saved trap pos" class="WFGraph (strict)"("Visible"=FALSE) -> ()  [unwired: 2 in, 2 out]
  n3329 = property on="Trap Delta Graph" class="WFGraph (strict)"("Visible"=TRUE) -> ()  [unwired: 2 in, 2 out]
  n3330 = node-c288(w113) -> ()  [unwired: 1 out]
  n3331 = local write "Trap pos"(FALSE ("Trap pos")) -> ()
  n3332 = disable-structure shown="Disabled" {
    disable-tunnel: w117 -> [w5242 _]
    disable-tunnel: w116 -> [w5241 _]
    frame Disabled {
      n3333 = VISA Close(VISA resource name=w5242, error in (no error)=w5241) -> (error out=w5243:errorcluster)
      n3334 = call <vilib>:"Simple Error Handler.vi"("error in (no error)"=w5243) -> ()  [unwired: 1 in, 8 out]
    }
    frame Enabled {
    }
  }
  n3335 = node-c288(w124) -> ()  [unwired: 1 out]
  n3336 = node-c288(w199) -> ()  [unwired: 1 out]
  n3337 = flat-sequence {
    tunnel: w290 -> [w5247]
    tunnel: w292 -> [w5248]
    tunnel: [w5246] -> w271
    tunnel: [w5245] -> w270
    tunnel: w255 -> [_]
    tunnel: w207 -> [_]
    tunnel: w130 -> [_]
    tunnel: w271 -> [w5249]
    tunnel: w270 -> [w5250]
    frame #0 {
      w5244 = FALSE ("AI to FIFO")
      n3338 = xnode "Read/Write Control"("FPGA VI Reference In"=w5248, "error in"=w5247, "AI to FIFO"=w5244, "APD to FIFO"=w5244) -> ("FPGA VI Reference Out"=w5246:T20, "error out"=w5245:errorcluster)
    }
    frame #1 {
      n3339 = xnode "Close FPGA VI Reference"("FPGA VI Reference In"=w5249, "error in"=w5250) -> ("error out"=→"error out":errorcluster)
    }
  }
